vi "UHR-Fleezers Control (host) - 10.8MV_trial2.vi"() -> ()   [LabVIEW 2010] (continued)
          tunnel: [w5180] -> w5154
          tunnel: w5153 -> [w5180]
          tunnel: [w5179] -> w5147
          tunnel: w5146 -> [w5179]
          tunnel: [w5178] -> w5139
          tunnel: w5138 -> [w5178]
          tunnel: [w5184] -> w5155
          tunnel: w5154 -> [w5184]
          tunnel: [w5183] -> w5148
          tunnel: w5147 -> [w5183]
          tunnel: [w5182] -> w5140
          tunnel: w5139 -> [w5182]
          tunnel: w5155 -> [w5190]
          tunnel: w5148 -> [w5189]
          tunnel: [w5187] -> w5141
          tunnel: w5140 -> [w5187]
          tunnel: w5141 -> [w5191]
          frame #0 {
            n1099 = local read "Green Laser ON/Interlacing"() -> (w5159:bool)
            n1100 = local read "Green laser mode"() -> (w5158:enum32{"Laser ON", "Laser OFF", "Interlace"})
            n1101 = local read "Green FB On/Off"() -> (w5157:bool)
          }
          frame #1 {
            n1102 = property on="Green FB On/Off" class="Bool (strict)"("Val(Sgnl)"=FALSE ("Value (Signaling)")) -> ()  [unwired: 2 in, 2 out]
          }
          frame #2 {
            n1103 = property on="Green Laser ON/Interlacing" class="Bool (strict)"("Val(Sgnl)"=TRUE ("Value (Signaling)")) -> ()  [unwired: 2 in, 2 out]
            n1104 = property on="Flip Green Filter" class="Bool (strict)"("Val(Sgnl)"=TRUE ("Value (Signaling)")) -> ()  [unwired: 2 in, 2 out]
            n1105 = property on="Green laser mode" class="RadioBtnsControl (strict)"("Val(Sgnl)"=enum32{"Laser ON", "Laser OFF", "Interlace"}."Laser ON" ("Value (Signaling)")) -> ()  [unwired: 2 in, 2 out]
          }
          frame #3 {
            n1106 = Wait (ms)(milliseconds to wait=u32 500) -> ()  [unwired: 1 out]
          }
          frame #4 {
            n1107 = property on="Confocal Image" class="Bool (strict)"("Val(Sgnl)"=TRUE ("Value (Signaling)")) -> ()  [unwired: 2 in, 2 out]
          }
          frame #5 {
            n1108 = Wait (ms)(milliseconds to wait=u32 2000) -> ()  [unwired: 1 out]
          }
          frame #6 {
            n1109 = while {
              stop <- w5185 stop-if-true
              n1110 = local read "Saving..."() -> (w5186:bool)
              n1111 = Not(x=w5186) -> (.not. x?=w5185:bool)
            }
          }
          frame #7 {
            n1112 = property on="Flip Green Filter" class="Bool (strict)"("Val(Sgnl)"=TRUE ("Value (Signaling)")) -> ()  [unwired: 2 in, 2 out]
            n1113 = property on="Green Laser ON/Interlacing" class="Bool (strict)"("Val(Sgnl)"=w5190) -> ()  [unwired: 2 in, 2 out]
            n1114 = property on="Green laser mode" class="RadioBtnsControl (strict)"("Val(Sgnl)"=w5189) -> ()  [unwired: 2 in, 2 out]
          }
          frame #8 {
            n1115 = property on="Green FB On/Off" class="Bool (strict)"("Val(Sgnl)"=w5191) -> ()  [unwired: 2 in, 2 out]
          }
        }
      }
      event "Stop All": Value Change {
        n1116 = event-data() -> ()  [unwired: 1 in, 5 out]
        n1117 = local read "Stop All"() -> (w5192:bool)
      }
    }
    n1118 = node-c288() -> ()  [unwired: 1 in, 1 out]
  }
  n1119 = node-c288() -> (w76:T26)  [unwired: 4 out]
  n1120 = timed-loop "Mouse control: trap position (AOM deflection), set confocal spot from image" {
    tunnel: [w5194] -> w34
    tunnel: w24 -> [w5193]
    timing: w76 -> [_]
    timing-out: [_] -> w75
    stop <- w5194 stop-if-true
    n1121 = node-c288() -> ()  [unwired: 2 out]
    n1122 = event shown="[0] \"Pane\": Mouse Down" {
      selector: _ -> [_ _]
      dyn-events: _ -> [_ _]
      timeout: _ -> [_ _]
      tunnel: w5193 -> [w5197 _]
      event Mouse Down {
        n1123 = event-data() -> ("Time"=w5199:u32, "Coords"=w5198:T7, "Button"=w5200:u16)  [unwired: 6 out]
        n1124 = case shown="1" w5200 {
          tunnel: w5199 -> [_ _ w5303]
          tunnel: w5198 -> [_ w5237 w5301]
          tunnel: w5197 -> [_ _ w5299]
          frame 0, Default {
          }
          frame 1 {
            n1125 = property on="APD 2" class="ImageControl"() -> ("Displayed Image Position"=w5207:cluster{"Left":i32, "Top":i32})  [unwired: 2 in, 2 out]
            n1126 = property on="APD 1" class="ImageControl"() -> ("Displayed Image Position"=w5236:cluster{"Left":i32, "Top":i32})  [unwired: 2 in, 2 out]
            n1127 = property on="Detection Laser X" class="ImageControl"() -> ("Displayed Image Position"=w5233:cluster{"Left":i32, "Top":i32})  [unwired: 2 in, 2 out]
            n1128 = property on="Detection Laser Y" class="ImageControl"() -> ("Displayed Image Position"=w5232:cluster{"Left":i32, "Top":i32})  [unwired: 2 in, 2 out]
            n1129 = property on="APD 2" class="ImageControl"() -> ("Displayed Image Size"=w5206:cluster{"Width":u32, "Height":u32})  [unwired: 2 in, 2 out]
            n1130 = property on="APD 1" class="ImageControl"() -> ("Displayed Image Size"=w5234:cluster{"Width":u32, "Height":u32})  [unwired: 2 in, 2 out]
            n1131 = property on="Detection Laser X" class="ImageControl"() -> ("Displayed Image Size"=w5235:cluster{"Width":u32, "Height":u32})  [unwired: 2 in, 2 out]
            n1132 = property on="Detection Laser Y" class="ImageControl"() -> ("Displayed Image Size"=w5231:cluster{"Width":u32, "Height":u32})  [unwired: 2 in, 2 out]
            n1133 = Unbundle By Name(w5206) -> ("Width"=w5203:u32, "Height"=w5202:u32)
            n1134 = Unbundle By Name(w5207) -> ("Left"=w5205:i32, "Top"=w5204:i32)
            n1135 = Unbundle By Name(w5234) -> ("Width"=w5228:u32, "Height"=w5227:u32)
            n1136 = Unbundle By Name(w5235) -> ("Width"=w5224:u32, "Height"=w5223:u32)
            n1137 = Unbundle By Name(w5231) -> ("Width"=w5220:u32, "Height"=w5219:u32)
            n1138 = Unbundle By Name(w5236) -> ("Left"=w5230:i32, "Top"=w5229:i32)
            n1139 = Unbundle By Name(w5233) -> ("Left"=w5226:i32, "Top"=w5225:i32)
            n1140 = Unbundle By Name(w5232) -> ("Left"=w5222:i32, "Top"=w5221:i32)
            n1141 = Bundle("Left"=w5205, "Top"=w5204, "Width"=w5203, "Height"=w5202) -> (w5201:T35)  [unwired: 1 in]
            n1142 = Bundle("Left"=w5230, "Top"=w5229, "Width"=w5228, "Height"=w5227) -> (w5218:T35)  [unwired: 1 in]
            n1143 = Bundle("Left"=w5226, "Top"=w5225, "Width"=w5224, "Height"=w5223) -> (w5217:T35)  [unwired: 1 in]
            n1144 = Bundle("Left"=w5222, "Top"=w5221, "Width"=w5220, "Height"=w5219) -> (w5216:T35)  [unwired: 1 in]
            n1145 = Build Cluster Array(w5201, w5218, w5217, w5216) -> (w5215:T36)
            n1146 = for {
              tunnel: w5237 -> [w5248]
              tunnel: w5215 -> [w5249] mode=indexing
              shift-right: [w5246] -> w5213
              shift-left: TRUE -> [w5247]
              shift-right: [w5245] -> w5211
              shift-left: _ -> [w5241]
              shift-right: [w5244] -> w5210
              shift-left: _ -> [w5240]
              shift-right: [w5243] -> w5209
              shift-left: _ -> [w5239]
              shift-right: [w5242] -> w5208
              shift-left: _ -> [w5238]
              n1147 = case shown="True" w5247 {
                selector: w5247 -> [w5254 _]
                tunnel: w5249 -> [_ w5263]
                tunnel: w5248 -> [_ w5261]
                tunnel: [w5254 w5259] -> w5246
                tunnel: [w5253 w5258] -> w5245
                tunnel: [w5252 w5257] -> w5244
                tunnel: [w5251 w5256] -> w5243
                tunnel: [w5250 w5255] -> w5242
                tunnel: w5241 -> [w5253 _]
                tunnel: w5240 -> [w5252 _]
                tunnel: w5239 -> [w5251 _]
                tunnel: w5238 -> [w5250 _]
                frame False {
                }
                frame True {
                  n1148 = Unbundle(w5263) -> (w5262:T35)
                  n1149 = call "isclickinwindow.vi"("Image Param"=w5262, "Point32"=w5261) -> ("4 Y"=w5255:i32, "3 Height"=w5256:i32, "2 X"=w5257:i32, "1 Width"=w5258:i32, "In image?"=w5260:bool)  [unwired: 1 in]
                  n1150 = Not(x=w5260) -> (.not. x?=w5259:bool)
                }
              }
            }
            n1151 = Not(x=w5213) -> (.not. x?=w5212:bool)
            n1152 = case shown="True" w5212 {
              tunnel: w5210 -> [_ w5276]
              tunnel: w5208 -> [_ w5275]
              tunnel: w5211 -> [_ w5274]
              tunnel: w5209 -> [_ w5273]
              frame False {
              }
              frame True {
                w5269 = FALSE ("Get Point")
                n1153 = local read "Scan lines (y)"() -> (w5278:u64)
                n1154 = local read "Actual MCL Inc (V)"() -> (w5270:dbl)
                n1155 = local read "Scan steps (MCL)"() -> (w5277:u64)
                n1156 = Divide "Y Pix/step"(x=w5273, y=w5278) -> (x/y=w5285:dbl)
                n1157 = Divide "Y V/pix"(x=w5270, y=w5285) -> (x/y=w5284:dbl)
                n1158 = Divide "Y half step offset"(x=w5270, y=2.0) -> (x/y=w5286:dbl)
                n1159 = Divide "X pix/step"(x=w5274, y=w5277) -> (x/y=w5283:dbl)
                n1160 = Negate(x=w5286) -> (-x=w5287:dbl)
                n1161 = local read "Initial Y"() -> (w5293:dbl)
                n1162 = Multiply(x=w5275, y=w5284) -> (x*y=w5294:dbl)
                n1163 = Divide "X half step offset"(x=w5270, y=2.0) -> (x/y=w5280:dbl)
                n1164 = Divide "X V/pix"(x=w5270, y=w5283) -> (x/y=w5282:dbl)
                n1165 = Multiply(x=w5270, y=w5277) -> (x*y=w5289:dbl)
                n1166 = Compound Arithmetic op=ADD(w5287, w5294, w5293) -> (w5271:dbl)
                "Pointer Y (V)" <- w5271
                n1167 = Multiply(x=w5282, y=w5276) -> (x*y=w5291:dbl)
                n1168 = Negate(x=w5280) -> (-x=w5279:dbl)
                n1169 = local read "Initial X"() -> (w5292:dbl)
                n1170 = Negate(x=w5291) -> (-x=w5290:dbl)
                n1171 = Compound Arithmetic op=ADD(w5279, w5289, w5292, w5290) -> (w5272:dbl)
                "Pointer X (V)" <- w5272
                n1172 = Or(x="Set X Only", y="Set Confocal Spot (X-Y)") -> (x .or. y?=w5265:bool)
                n1173 = Or(x="Set Confocal Spot (X-Y)", y="Set Y Only") -> (x .or. y?=w5264:bool)
                n1174 = case shown="True" w5265 {
                  tunnel: w5272 -> [_ w5295]
                  frame False {
                  }
                  frame True {
                    n1175 = property on="AO2" class="Slide (strict)"("Val(Sgnl)"=w5295) -> ()  [unwired: 2 in, 2 out]
                  }
                }
                n1176 = case shown="True" w5264 {
                  tunnel: w5271 -> [_ w5296]
                  frame False {
                  }
                  frame True {
                    n1177 = property on="AO1" class="Slide (strict)"("Val(Sgnl)"=w5296) -> ()  [unwired: 2 in, 2 out]
                  }
                }
                n1178 = local write "Set Confocal Spot (X-Y)"(w5269) -> ()
                n1179 = local write "Set X Only"(w5269) -> ()
                n1180 = local write "Set Y Only"(w5269) -> ()
              }
            }
          }
          frame 3 {
            n1181 = local read "BD 2 Frequency 1 (MHz)"() -> (w5297:dbl)
            n1182 = local read "BD 1 Frequency 1 (MHz)"() -> (w5298:dbl)
            n1183 = local write "Manipulating Trap"(TRUE ("Manipulating Trap")) -> ()
            n1184 = local write "Coords"(T7 {"Horizontal"=0, "Vertical"=0} ("Coords")) -> ()
            n1185 = while {
              tunnel: w5303 -> [w5308]
              tunnel: w5301 -> [w5307]
              tunnel: w5299 -> [w5306]
              tunnel: w5298 -> [w5305]
              tunnel: w5297 -> [w5304]
              stop <- w5309 stop-if-true
              n1186 = event shown="[0] \"Pane\": Mouse Move" {
                selector: _ -> [_ _]
                dyn-events: _ -> [_ _]
                timeout: _ -> [_ _]
                tunnel: ["Force Manip Abort" w5373] -> w5309
                tunnel: w5308 -> [w5316 _]
                tunnel: w5307 -> [w5314 _]
                tunnel: w5306 -> [w5313 _]
                tunnel: w5305 -> [w5312 _]
                tunnel: w5304 -> [w5311 _]
                event Mouse Move {
                  n1187 = event-data() -> ("Time"=w5317:u32, "Coords"=w5318:T7)  [unwired: 3 out]
                  n1188 = Less?(x=w5317, y=w5316) -> (x < y?=w5315:bool)
                  n1189 = case "Makes sure old motion events prior to mouse click aren't used" shown="False" w5315 {
                    tunnel: w5318 -> [w5360 _]
                    tunnel: w5314 -> [w5361 _]
                    tunnel: w5313 -> [w5338 _]
                    tunnel: w5312 -> [w5334 _]
                    tunnel: w5311 -> [w5333 _]
                    frame False {
                      n1190 = Subtract(x=w5360, y=w5361) -> (x-y=w5359:T7)
                      "Coords" <- w5359
                      n1191 = local read "Y RF Frequency Limits (MHz)"() -> (w5319:T16)
                      n1192 = To Double Precision Float(number=w5359) -> (double precision float=w5358:cluster{"Horizontal":dbl, "Vertical":dbl})
                      n1193 = Multiply(x=cluster{"Horizontal":dbl, "Vertical":dbl} {"Horizontal"=-1.0, "Vertical"=1.0}, y="Manipulation Scaling") -> (x*y=w5354:cluster{"Horizontal":dbl, "Vertical":dbl})
                      n1194 = local read "X RF Frequency Limits (MHz)"() -> (w5320:T16)
                      n1195 = Multiply(x=w5358, y=w5354) -> (x*y=w5356:cluster{"Horizontal":dbl, "Vertical":dbl})
                      n1196 = Unbundle By Name(w5356) -> ("Horizontal"=w5351:dbl, "Vertical"=w5355:dbl)
                      n1197 = Unbundle By Name(w5319) -> ("Maximum"=w5322:dbl, "Minimum"=w5321:dbl)
                      n1198 = Boolean To (0,1)(Boolean="Manip. X?") -> (0, 1=w5349:i16)
                      n1199 = Boolean To (0,1)(Boolean="Manip. Y?") -> (0, 1=w5346:i16)
                      n1200 = local read "BD 1 Frequency 2 (MHz)"() -> (w5336:dbl)
                      n1201 = Multiply(x=w5355, y=w5346) -> (x*y=w5348:dbl)
                      n1202 = Multiply(x=w5349, y=w5351) -> (x*y=w5352:dbl)
                      n1203 = local read "BD 2 Frequency 2 (MHz)"() -> (w5335:dbl)
                      n1204 = Unbundle By Name(w5320) -> ("Maximum"=w5324:dbl, "Minimum"=w5323:dbl)
                      n1205 = Add(x=w5333, y=w5348) -> (x+y=w5326:dbl)
                      n1206 = Add(x=w5334, y=w5352) -> (x+y=w5328:dbl)
                      n1207 = In Range and Coerce(upper limit=w5324, x=w5328, lower limit=w5323) -> (coerced(x)=w5327:dbl)  [unwired: 1 out]
                      n1208 = In Range and Coerce(upper limit=w5322, x=w5326, lower limit=w5321) -> (coerced(x)=w5325:dbl)  [unwired: 1 out]
                      n1209 = Subtract(x=w5327, y=w5336) -> (x-y=w5345:dbl)
                      n1210 = Subtract(x=w5325, y=w5335) -> (x-y=w5344:dbl)
                      n1211 = Square(x=w5345) -> (x^2=w5343:dbl)
                      n1212 = Square(x=w5344) -> (x^2=w5342:dbl)
                      n1213 = Add(x=w5343, y=w5342) -> (x+y=w5341:dbl)
                      n1214 = Square Root(x=w5341) -> (sqrt(x)=w5337:dbl)
                      n1215 = In Range and Coerce(upper limit="Limit Max (MHz)", x=w5337, lower limit="Limit Min (MHz)") -> (In Range?=w5330:bool)  [unwired: 1 out]
                      n1216 = Not(x="Limits Enable") -> (.not. x?=w5329:bool)
                      n1217 = Or(x=w5330, y=w5329) -> (x .or. y?=w5331:bool)
                      n1218 = case shown="True" w5331 {
                        tunnel: w5338 -> [_ w5371]
                        tunnel: w5337 -> [_ w5362]
                        tunnel: w5327 -> [_ w5369]
                        tunnel: w5336 -> [_ w5368]
                        tunnel: w5325 -> [_ w5367]
                        tunnel: w5335 -> [_ w5366]
                        tunnel: w5320 -> [_ w5364]
                        tunnel: w5319 -> [_ w5363]
                        frame False {
                        }
                        frame True {
                          n1219 = local read "BD 1 Frequency 3 (MHz)"() -> (w5370:dbl)
                          n1220 = local read "BD 2 Frequency 3 (MHz)"() -> (w5365:dbl)
                          n1221 = local write "Trap Delta (MHz)"(w5362) -> ()
                          n1222 = property on="Initial delta (MHz)" class="DigNum (strict)"("Val(Sgnl)"=w5362) -> ()  [unwired: 2 in, 2 out]
                          n1223 = call "set RF board frequency - interlace.vi"("Board 2 Frequency Limits"=w5363, "Board 1 Frequency Limits"=w5364, "FPGA VI Reference In"=w5371, "Board 2 Frequency 3 (MHz)"=w5365, "Board 1 Frequency 3 (MHz)"=w5370, "Board 2 Frequency 2 (MHz)"=w5366, "Board 2 Frequency 1 (MHz)"=w5367, "Board 1 Frequency 2 (MHz)"=w5368, "Board 1 Frequency 1  (MHz)"=w5369) -> ()  [unwired: 1 in, 2 out]
                          n1224 = local write "BD 2 Frequency 1 (MHz)"(w5367) -> ()
                          n1225 = local write "BD 1 Frequency 1 (MHz)"(w5369) -> ()
                        }
                      }
                    }
                    frame True {
                    }
                  }
                }
                event Mouse Up {
                  n1226 = event-data() -> ("Button"=w5372:u16)  [unwired: 8 out]
                  n1227 = case shown="3" w5372 {
                    tunnel: [FALSE TRUE] -> w5373
                    frame 0, Default {
                    }
                    frame 3 {
                      n1228 = local write "Manipulating Trap"(FALSE ("Manipulating Trap")) -> ()
                    }
                  }
                }
              }
            }
          }
        }
      }
      event Mouse Move {
        n1229 = event-data() -> ()  [unwired: 6 out]
      }
    }
    n1230 = local read "Stop All"() -> (w5194:bool)
    n1231 = node-c288() -> ()  [unwired: 2 out]
  }
  n1232 = node-c288(i64 1 ("Period"), 1 ("Processor")) -> (w164:T26)  [unwired: 2 out]
  n1233 = timed-loop "Acquire Data" {
    tunnel: w24 -> [w5631]
    tunnel: w40 -> [w5630]
    tunnel: [w5661] -> w33
    tunnel: [w5655] -> w32
    timing: w164 -> [_]
    timing-out: [_] -> w163
    tunnel: w59 -> [w5459]
    stop <- "Stop All" stop-if-true
    (unwired) u32 0 ("Number of Elements")
    w5446 = "NI_ChannelName" ("name")
    n1234 = node-c288() -> ()  [unwired: 2 out]
    n1235 = First Call?() -> (First Call?: T/F=w5412:bool)
    n1236 = Or(x="Reset", y=w5412) -> (x .or. y?=w5413:bool)
    n1237 = case "Reset data stream" shown="True" w5413 {
      tunnel: w5631 -> [w5749 w5757]
      tunnel: w5630 -> [w5748 w5756]
      tunnel: [w5749 w5751] -> w5626
      tunnel: [w5748 w5750] -> w5625
      frame False {
      }
      frame True {
        w5754 = TRUE ("AI to FIFO")
        n1238 = local write "Overflow (data lost)"(FALSE ("Overflow (data lost)")) -> ()
        n1239 = call "reset FPGA DMA.vi"("error in"=w5756, "FPGA VI Reference In"=w5757) -> ("error out"=w5752:errorcluster, "FPGA VI Reference Out"=w5753:T19)
        n1240 = xnode "Read/Write Control"("FPGA VI Reference In"=w5753, "error in"=w5752, "AI to FIFO"=w5754, "APD to FIFO"=w5754) -> ("FPGA VI Reference Out"=w5751:T19, "error out"=w5750:errorcluster)
      }
    }
    n1241 = Or(x="Start AOD Scan", y="Trap Raster Scan") -> (x .or. y?=w5576:bool)
    n1242 = case "Start AOM raster scan" shown="True" w5576 {
      tunnel: w5626 -> [w7357 w7367]
      tunnel: w5625 -> [w7356 w7366]
      tunnel: [w7357 w7360] -> w5624
      tunnel: [w7356 w7359] -> w5623
      frame False {
      }
      frame True {
        n1243 = case shown="True" "Restart DMA? (AOD)" {
          tunnel: [w7778 w7780] -> w7361
          tunnel: [w7777 w7779] -> w7362
          tunnel: w7367 -> [w7778 w7782]
          tunnel: w7366 -> [w7777 w7781]
          frame False {
          }
          frame True {
            n1244 = local write "Overflow (data lost)"(FALSE ("Overflow (data lost)")) -> ()
            n1245 = call "reset FPGA DMA.vi"("error in"=w7781, "FPGA VI Reference In"=w7782) -> ("error out"=w7779:errorcluster, "FPGA VI Reference Out"=w7780:T19)
          }
        }
        n1246 = local write "Trap Raster Scan"(FALSE ("Trap Raster Scan")) -> ()
        n1247 = case shown="False" "Move MCL Also?" {
          tunnel: w7362 -> [w7370 w7479]
          tunnel: w7361 -> [w7371 w7480]
          tunnel: [w7369 w7483] -> w7360
          tunnel: [w7368 w7482] -> w7359
          frame False {
            w7372 = TRUE ("AI to FIFO")
            n1248 = xnode "Read/Write Control"("FPGA VI Reference In"=w7371, "error in"=w7370, "AI to FIFO"=w7372, "APD to FIFO"=w7372, "Start scan"=w7372) -> ("FPGA VI Reference Out"=w7369:T19, "error out"=w7368:errorcluster)
          }
          frame True {
            w7476 = FALSE ("1D or 2D Scan?")
            w7481 = TRUE ("AI to FIFO")
            # "Count for MCL loop"
            # "N total cycles"
            # "N steps"
            # "V_int"
            n1249 = local read "Scan Range (nm)"() -> (w7458:dbl)
            n1250 = local read "Number of F/B Scans (AOD)"() -> (w7475:u16)
            n1251 = Sign(1:w7458) -> (0:w7457:dbl)
            n1252 = Compound Arithmetic op=MULTIPLY(w7458, "MCL Step Position Ratio", "MCL/AOM Scale Tweak") -> (w7462:dbl)
            n1253 = Negate(x=w7457) -> (-x=w7454:dbl)
            n1254 = Multiply(x=w7454, y="MCL Step Increment (V_int)") -> (x*y=w7456:dbl)
            n1255 = Divide(x=w7462, y="MCL X Cal (nm/V)") -> (x/y=w7468:dbl)
            n1256 = Multiply(x=32767.0 ("y"), y=w7468) -> (x*y=w7474:dbl)
            n1257 = local read "Total Counts (ticks)"() -> (w7459:u32)
            n1258 = local read "Cycles/step (AOD)"() -> (w7470:u64)
            n1259 = local read "Scan steps (AOD)"() -> (w7471:u64)
            n1260 = Divide(x=w7474, y=10.0) -> (x/y=w7467:dbl)
            n1261 = Divide(x=w7467, y="MCL Step Increment (V_int)") -> (x/y=w7465:dbl)
            n1262 = Absolute Value(x=w7465) -> (abs(x)=w7453:dbl)
            n1263 = Compound Arithmetic op=MULTIPLY(w7471, w7470, w7459) -> (w7466:u64)
            n1264 = local write "wait to reset values"(w7481) -> ()
            n1265 = local write "MCL Scanning"(w7481) -> ()
            n1266 = Divide(x=w7466, y=w7453) -> (x/y=w7463:dbl)
            "MCL Count" <- w7463
            n1267 = xnode "Read/Write Control"("FPGA VI Reference In"=w7480, "error in"=w7479, "Scan steps (MCL)"=w7453, "Number of scans (MCL)"=w7475, "Cycles per step (MCL)"=u64 1, "Scan freq.  increment (MCL)"=w7456, "1D or 2D Scan?"=w7476, "MCL Scan Axis"=w7476, "Cont. Scan (MCL)"=w7476, "MCL count"=w7463) -> ("FPGA VI Reference Out"=w7478:T19, "error out"=w7477:errorcluster)
            n1268 = xnode "Read/Write Control"("FPGA VI Reference In"=w7478, "error in"=w7477, "AI to FIFO"=w7481, "APD to FIFO"=w7481, "Start scan"=w7481, "Start scan (MCL)"=w7481) -> ("FPGA VI Reference Out"=w7483:T19, "error out"=w7482:errorcluster)
          }
        }
        "Raster Scanning..." <- TRUE ("Scanning...")
      }
    }
    n1269 = And(x="Save scans", y=w5576) -> (x .and. y?=w5622:bool)
    n1270 = Compound Arithmetic op=OR("Start MCL Scan", "Confocal Image", "Confocal Linescan") -> (w5574:bool)
    n1271 = And(x="Save Data (MCL)", y=w5574) -> (x .and. y?=w5621:bool)
    n1272 = case "Start MCL raster scan" shown="True" w5574 {
      tunnel: w5624 -> [w6634 w6649]
      tunnel: w5623 -> [w6633 w6648]
      tunnel: [w6634 w6644] -> w5381
      tunnel: [w6633 w6643] -> w5380
      tunnel: [FALSE w6642] -> w5607
      tunnel: "Start MCL Scan" -> [_ w6637]
      tunnel: "Confocal Image" -> [_ w6636]
      tunnel: "Confocal Linescan" -> [_ _]
      frame False {
      }
      frame True {
        w6642 = TRUE
        n1273 = case shown="True" "Restart DMA? (MCL)" {
          tunnel: [w6894 w6896] -> w6647
          tunnel: [w6893 w6895] -> w6646
          tunnel: w6649 -> [w6894 w6899]
          tunnel: w6648 -> [w6893 w6898]
          frame False {
          }
          frame True {
            n1274 = call "reset FPGA DMA.vi"("error in"=w6898, "FPGA VI Reference In"=w6899) -> ("error out"=w6895:errorcluster, "FPGA VI Reference Out"=w6896:T19)
            n1275 = local write "Overflow (data lost)"(FALSE ("Overflow (data lost)")) -> ()
          }
        }
        n1276 = case shown="False" w6637 {
          selector: w6637 -> [_ w6653]
          tunnel: w6636 -> [w6652 _]
          tunnel: [w6652 w6653] -> w6635
          frame False {
            n1277 = property on="2D or 1D Scan" class="Bool (strict)"("Val(Sgnl)"=w6652) -> ()  [unwired: 2 in, 2 out]
            n1278 = property on="Confocal Image" class="Bool (strict)"("Value"=FALSE ("Start Confocal Map")) -> ()  [unwired: 2 in, 2 out]
          }
          frame True {
          }
        }
        n1279 = local write "MCL Scanning"(w6642) -> ()
        n1280 = local read "AO1"() -> (w6639:dbl)
        n1281 = local read "AO2"() -> (w6638:dbl)
        n1282 = case shown="True" "Center Scan" {
          tunnel: w6647 -> [w6660 w6772]
          tunnel: w6646 -> [w6659 w6771]
          tunnel: [w6658 w6770] -> w6644
          tunnel: [w6657 w6769] -> w6643
          tunnel: [w6655 w6756] -> w6641
          tunnel: [w6654 w6755] -> w6640
          tunnel: w6639 -> [w6655 w6761]
          tunnel: w6638 -> [w6654 w6764]
          tunnel: w6635 -> [_ _]
          frame False {
            w6656 = TRUE ("AI to FIFO")
            n1283 = xnode "Read/Write Control"("FPGA VI Reference In"=w6660, "error in"=w6659, "AI to FIFO"=w6656, "APD to FIFO"=w6656, "Start scan (MCL)"=w6656) -> ("FPGA VI Reference Out"=w6658:T19, "error out"=w6657:errorcluster)
          }
          frame True {
            w6768 = TRUE ("AI to FIFO")
            n1284 = local read "Scan steps (MCL)"() -> (w6747:u64)
            n1285 = local read "Scan lines (y)"() -> (w6743:u64)
            n1286 = local read "Fast Scan Dir"() -> (w6754:bool)
            n1287 = local read "Actual MCL Inc (V)"() -> (w6744:dbl)
            n1288 = Decrement(x=w6743) -> (x-1=w6742:u64)
            n1289 = Decrement(x=w6747) -> (x-1=w6746:u64)
            n1290 = Multiply(x=w6744, y=w6742) -> (x*y=w6741:dbl)
            n1291 = Divide(x=w6741, y=2.0) -> (x/y=w6751:dbl)
            n1292 = Multiply(x=w6744, y=w6746) -> (x*y=w6745:dbl)
            n1293 = Divide(x=w6745, y=2.0) -> (x/y=w6750:dbl)
            n1294 = Select(t=w6750, s=w6754, f=w6751) -> (s? t:f=w6749:dbl)
            n1295 = Select(t=w6751, s=w6754, f=w6750) -> (s? t:f=w6753:dbl)
            n1296 = Subtract(x=w6761, y=w6753) -> (x-y=w6752:dbl)
            n1297 = Subtract(x=w6764, y=w6749) -> (x-y=w6748:dbl)
            n1298 = local read "2D or 1D Scan"() -> (w6766:bool)
            n1299 = Not(x=w6754) -> (.not. x?=w6760:bool)
            n1300 = Not(x=w6766) -> (.not. x?=w6762:bool)
            n1301 = And(x=w6754, y=w6762) -> (x .and. y?=w6763:bool)
            n1302 = And(x=w6762, y=w6760) -> (x .and. y?=w6765:bool)
            n1303 = Select(t=w6764, s=w6765, f=w6748) -> (s? t:f=w6755:dbl)
            n1304 = Select(t=w6761, s=w6763, f=w6752) -> (s? t:f=w6756:dbl)
            n1305 = call "Volt to I16.vi"("Voltage In"=w6756) -> ("I16 Voltage Out"=w6759:i16)
            n1306 = call "Volt to I16.vi"("Voltage In"=w6755) -> ("I16 Voltage Out"=w6758:i16)
            n1307 = xnode "Read/Write Control"("FPGA VI Reference In"=w6772, "error in"=w6771, "AI to FIFO"=w6768, "APD to FIFO"=w6768, "Start scan (MCL)"=w6768, "AO1"=w6759, "AO2"=w6758) -> ("FPGA VI Reference Out"=w6770:T19, "error out"=w6769:errorcluster)
          }
        }
        "Initial Y" <- w6641
        "Initial X" <- w6640
        "wait to reset values" <- w6642
      }
    }
    n1308 = local read "Trap Pos Elements/DMA read"() -> (w5455:u32)
    n1309 = local read "Trap AI Elements/DMA read"() -> (w5379:u32)
    n1310 = local read "APD Elements/DMA read"() -> (w5498:u32)
    n1311 = local read "Trap AI FIFO Depth"() -> (w5671:u32)
    n1312 = xnode "Invoke Method"("FPGA VI Reference In"=w5381, "error in"=w5380, "Number of Elements"=w5455, "Timeout (ms)"=-1) -> ("Data"=w5419:u16[], "Elements Remaining"=→"Trap Pos FIFO El Remaining":u32)  [unwired: 2 out]
    n1313 = xnode "Invoke Method"("FPGA VI Reference In"=w5381, "error in"=w5380, "Number of Elements"=w5379, "Timeout (ms)"=-1 ("Timeout")) -> ("FPGA VI Reference Out"=w5383:T19, "error out"=w5382:errorcluster, "Data"=w5378:i16[], "Elements Remaining"=w5384:u32)
    "Trap AI FIFO El. Rem." <- w5384
    n1314 = xnode "Get APD Data"("FPGA VI Reference In"=w5381, "error in"=w5380, "Number of Elements"=w5498, "Timeout (ms)"=-1) -> ("Data"=w5497:u32[], "Elements Remaining"=→"APD FIFO Elements Remaining":u32)  [unwired: 2 out]
    n1315 = Subtract(x=w5671, y=w5379) -> (x-y=w5670:u32)
    n1316 = Decimate 1D Array(w5419) -> (w5416:u16[], w5418:u16[], w5417:u16[])
    n1317 = Divide(x=w5384, y=w5670) -> (x/y=w5669:dbl)
    "Buffer Status" <- w5669
    n1318 = To Unsigned Long Integer(number=w5416) -> (unsigned 32bit integer=w5415:u32[])
    n1319 = Join Numbers(hi=w5418, lo=w5417) -> ((hi.lo)=w5414:u32[])
    n1320 = Equal?(x=w5669, y=1.0) -> (x = y?=w5667:bool)
    n1321 = Join Numbers(hi=w5415, lo=w5414) -> ((hi.lo)=w5408:u64[])
    n1322 = call "IR AOM word to freq - vec.vi"("Frequency Word In (double vec)"=w5408) -> ("Frequency Out"=w5454:dbl[])
    n1323 = case "Alert buffer overflow" shown="True" w5667 {
      frame False {
      }
      frame True {
        n1324 = call <vilib>:"Beep.vi"() -> ()  [unwired: 3 in, 9 out]
        "Overflow (data lost)" <- TRUE ("Overflow (data lost)")
      }
    }
    n1325 = Decimate 1D Array(w5454) -> (w5453:dbl[], w5452:dbl[])
    n1326 = Array Size(array=w5378) -> (size(s)=→"Waveform Chart":i32)
    n1327 = Build Array(w5453, w5452) -> (w5451:dbl[][])
    n1328 = local read "Trap Sets"() -> (w5535:u32)
    n1329 = case "Deinterlace trap data, average down PSD" shown="2" w5535 {
      tunnel: w5378 -> [w6929 w6994]
      tunnel: [w6926 w6991] -> w5528
      tunnel: [w6929 w6993] -> w5411
      tunnel: "Detector Type" -> [w6928 w6989]
      tunnel: [w6927 w6992] -> w5527
      tunnel: [w6925 w6990] -> w5642
      frame 1, Default {
        n1330 = Divide(x=w6929, y=3276.7) -> (x/y=w6930:dbl[])
        n1331 = Decimate 1D Array(w6930) -> (w6939:dbl[], w6938:dbl[], w6937:dbl[], w6936:dbl[], w6935:dbl[], w6934:dbl[], w6933:dbl[], w6932:dbl[])
        n1332 = case shown="\"IR-QPD + PSD + FB-QPD position\"" w6928 {
          tunnel: w6939 -> [w6963 w6988]
          tunnel: w6938 -> [w6962 w6987]
          tunnel: w6937 -> [w6947 w6965]
          tunnel: w6936 -> [w6948 w6975]
          tunnel: w6935 -> [w6961 w6986]
          tunnel: w6934 -> [w6960 w6985]
          tunnel: w6933 -> [w6944 w6966]
          tunnel: w6932 -> [w6943 w6964]
          tunnel: [w6942 w6972] -> w6927
          tunnel: [w6941 w6971] -> w6926
          tunnel: [w6940 w6970] -> w6925
          frame "IR-QPD + PSD + FB-QPD", Default {
            w6940 = 0  # Channel pattern
            n1333 = Divide(x=w6963, y=w6948) -> (x/y=w6950:dbl[])
            n1334 = Divide(x=w6962, y=w6948) -> (x/y=w6949:dbl[])
            n1335 = Divide(x=w6961, y=w6944) -> (x/y=w6946:dbl[])
            n1336 = Divide(x=w6960, y=w6943) -> (x/y=w6945:dbl[])
            n1337 = Build Array(w6950, w6949, w6948, w6947, w6946, w6945, w6944, w6943) -> (w6941:dbl[][])
            n1338 = Bundle("T1 Y", "T1 X", "T1 Sum", "FB Sum", "PSD Y", "PSD X", "PSD Y Sum", "PSD X Sum") -> (w6959:T44)  [unwired: 1 out]
            n1339 = Cluster To Array(cluster=w6959) -> (array=w6942:string[])
          }
          frame "IR-QPD + PSD + FB-QPD position" {
            w6970 = 3  # Channel pattern
            n1340 = Negate(x=w6966) -> (-x=w6967:dbl[])
            n1341 = Divide(x=w6988, y=w6975) -> (x/y=w6977:dbl[])
            n1342 = Divide(x=w6987, y=w6975) -> (x/y=w6976:dbl[])
            n1343 = Divide(x=w6986, y=w6966) -> (x/y=w6974:dbl[])
            n1344 = Divide(x=w6985, y=w6967) -> (x/y=w6973:dbl[])
            n1345 = Build Array(w6977, w6976, w6975, w6964, w6965, w6974, w6973, w6966) -> (w6971:dbl[][])
            n1346 = Bundle("T1 Y", "T1 X", "T1 Sum", "FB X", "FB Sum", "PSD Y", "PSD X", "PSD Y Sum") -> (w6984:T44)  [unwired: 1 out]
            n1347 = Cluster To Array(cluster=w6984) -> (array=w6972:string[])
          }
        }
      }
      frame 2 {
        n1348 = case shown="\"UCB Fleezers 052511\"" w6989 {
          tunnel: w6994 -> [w7056 w7123 w7151 w7258]
          tunnel: [w6995 w7115 w7146 w7189] -> w6993
          tunnel: [w7022 w7106 w7148 w7236] -> w6992
          tunnel: [w7021 w7070 w7125 w7203] -> w6991
          tunnel: [w7015 w7105 w7188 w7234] -> w6990
          frame "IR-QPD + PSD + FB-QPD", Default {
            w7015 = 1  # Channel pattern
            # "time average x2 the 4th signal and the 4 psd signals (detection laser)"
            # "deinterlace 3 signals from qpd"
            n1349 = Decimate 1D Array(w7056) -> (w7055:i16[], w7054:i16[], w7020:i16[], w7053:i16[], w7043:i16[], w7041:i16[], w7040:i16[], w7038:i16[])
            n1350 = call "downsample 1D array - double.vi"("Ave N"=2.0, "Array In"=w7043) -> ("Array Out"=w7042:dbl[])  [unwired: 1 out]
            n1351 = call "downsample 1D array - double.vi"("Ave N"=2.0, "Array In"=w7038) -> ("Array Out"=w7037:dbl[])  [unwired: 1 out]
            n1352 = call "downsample 1D array - double.vi"("Ave N"=2.0, "Array In"=w7040) -> ("Array Out"=w7039:dbl[])  [unwired: 1 out]
            n1353 = call "downsample 1D array - double.vi"("Ave N"=2.0, "Array In"=w7041) -> ("Array Out"=w7023:dbl[])  [unwired: 1 out]
            n1354 = Decimate 1D Array(w7055) -> (w7052:i16[], w7024:i16[])
            n1355 = Decimate 1D Array(w7054) -> (w7051:i16[], w7049:i16[])
            n1356 = Decimate 1D Array(w7053) -> (w7050:i16[], w7048:i16[])
            n1357 = Decimate 1D Array(w7020) -> (w7019:i16[], w7018:i16[])
            n1358 = Interleave 1D Arrays(w7052, w7051, w7050, w7024, w7049, w7048, w7019, w7018, w7042, w7023, w7039, w7037) -> (w7036:dbl[])
            n1359 = To Word Integer(number=w7036) -> (16bit integer=w6995:i16[])
            n1360 = Divide(x=w7036, y=3276.7) -> (x/y=w7035:dbl[])
            n1361 = Decimate 1D Array(w7035) -> (w7034:dbl[], w7033:dbl[], w7032:dbl[], w7031:dbl[], w7030:dbl[], w7029:dbl[], w7017:dbl[], w7016:dbl[], w7028:dbl[], w7027:dbl[], w7026:dbl[], w7025:dbl[])
            n1362 = Divide(x=w7034, y=w7032) -> (x/y=w7002:dbl[])
            n1363 = Divide(x=w7033, y=w7032) -> (x/y=w7001:dbl[])
            n1364 = Divide(x=w7031, y=w7029) -> (x/y=w7000:dbl[])
            n1365 = Divide(x=w7030, y=w7029) -> (x/y=w6999:dbl[])
            n1366 = Divide(x=w7028, y=w7026) -> (x/y=w6998:dbl[])
            n1367 = Divide(x=w7027, y=w7025) -> (x/y=w6997:dbl[])
            n1368 = Bundle("T1 Y", "T1 X", "T1 Sum", "T2 Y", "T2 X", "T2 Sum", "T1 FB Sum", "T2 FB Sum", "PSD Y", "PSD X", "PSD Y Sum", "PSD X Sum") -> (w7003:T45)  [unwired: 1 out]
            n1369 = Build Array(w7002, w7001, w7032, w7000, w6999, w7029, w7017, w7016, w6998, w6997, w7026, w7025) -> (w7021:dbl[][])
            n1370 = Cluster To Array(cluster=w7003) -> (array=w7022:string[])
          }
          frame "IR-QPD + PSD + FB-QPD X position" {
            w7105 = 2  # Channel pattern
            # "convert\nADC numbers\nto volts"
            # "time average x2 the 3 psd signals (detection laser)"
            # "deinterlace 3 signals from qpds"
            n1371 = Decimate 1D Array(w7123) -> (w7122:i16[], w7121:i16[], w7058:i16[], w7059:i16[], w7068:i16[], w7065:i16[], w7062:i16[], w7093:i16[])
            n1372 = Decimate 1D Array(w7122) -> (w7120:i16[], w7107:i16[])
            n1373 = call "downsample 1D array - I16.vi"("Ave N"=2.0, "Array In"=w7068) -> ("Array Out"=w7066:i16[])  [unwired: 1 in]
            n1374 = call "downsample 1D array - I16.vi"("Ave N"=2.0, "Array In"=w7065) -> ("Array Out"=w7063:i16[])  [unwired: 1 in]
            n1375 = Decimate 1D Array(w7121) -> (w7119:i16[], w7117:i16[])
            n1376 = Decimate 1D Array(w7059) -> (w7118:i16[], w7116:i16[])
            n1377 = Decimate 1D Array(w7093) -> (w7092:i16[], w7090:i16[])
            n1378 = Decimate 1D Array(w7058) -> (w7091:i16[], w7089:i16[])
            n1379 = call "downsample 1D array - I16.vi"("Ave N"=2.0, "Array In"=w7062) -> ("Array Out"=w7060:i16[])  [unwired: 1 in]
            n1380 = Interleave 1D Arrays(w7120, w7119, w7118, w7107, w7117, w7116, w7092, w7091, w7090, w7089, w7066, w7063, w7060) -> (w7115:i16[])
            n1381 = Divide(x=w7115, y=3276.7) -> (x/y=w7114:dbl[])
            n1382 = Decimate 1D Array(w7114) -> (w7113:dbl[], w7112:dbl[], w7111:dbl[], w7110:dbl[], w7109:dbl[], w7108:dbl[], w7081:dbl[], w7079:dbl[], w7078:dbl[], w7076:dbl[], w7075:dbl[], w7074:dbl[], w7071:dbl[])
            n1383 = Divide(x=w7113, y=w7111) -> (x/y=w7097:dbl[])
            n1384 = Divide(x=w7112, y=w7111) -> (x/y=w7096:dbl[])
            n1385 = Divide(x=w7110, y=w7108) -> (x/y=w7095:dbl[])
            n1386 = Divide(x=w7109, y=w7108) -> (x/y=w7094:dbl[])
            n1387 = Divide(x=w7081, y=w7079) -> (x/y=w7080:dbl[])
            n1388 = Divide(x=w7078, y=w7076) -> (x/y=w7077:dbl[])
            n1389 = Divide(x=w7075, y=w7071) -> (x/y=w7073:dbl[])
            n1390 = Negate(x=w7071) -> (-x=w7069:dbl[])
            n1391 = Divide(x=w7074, y=w7069) -> (x/y=w7072:dbl[])
            n1392 = Bundle("T1 Y", "T1 X", "T1 Sum", "T2 Y", "T2 X", "T2 Sum", "T1 FB X", "T1 FB Sum", "T2 FB X", "T2 FB Sum", "PSD Y", "PSD X", "PSD Y Sum") -> (w7098:T46)  [unwired: 1 out]
            n1393 = Build Array(w7097, w7096, w7111, w7095, w7094, w7108, w7080, w7079, w7077, w7076, w7073, w7072, w7071) -> (w7070:dbl[][])
            n1394 = Cluster To Array(cluster=w7098) -> (array=w7106:string[])
          }
          frame "UCB Fleezers 052511" {
            w7188 = 2  # Channel pattern
            n1395 = Decimate 1D Array(w7151) -> (w7186:i16[], w7185:i16[], w7150:i16[], w7149:i16[], w7143:i16[], w7140:i16[], w7139:i16[], w7138:i16[])
            n1396 = Decimate 1D Array(w7186) -> (w7184:i16[], w7169:i16[])
            n1397 = Decimate 1D Array(w7185) -> (w7183:i16[], w7181:i16[])
            n1398 = Decimate 1D Array(w7150) -> (w7182:i16[], w7180:i16[])
            n1399 = Decimate 1D Array(w7149) -> (w7145:i16[], w7144:i16[])
            n1400 = Decimate 1D Array(w7143) -> (w7142:i16[], w7141:i16[])
            n1401 = call "downsample 1D array - I16.vi"("Ave N"=2.0, "Array In"=w7140) -> ("Array Out"=w7137:i16[])  [unwired: 1 in]
            n1402 = call "downsample 1D array - I16.vi"("Ave N"=2.0, "Array In"=w7139) -> ("Array Out"=w7136:i16[])  [unwired: 1 in]
            n1403 = call "downsample 1D array - I16.vi"("Ave N"=2.0, "Array In"=w7138) -> ("Array Out"=w7135:i16[])  [unwired: 1 in]
            n1404 = Interleave 1D Arrays(w7184, w7183, w7182, w7169, w7181, w7180, w7145, w7142, w7144, w7141, w7137, w7136, w7135) -> (w7146:i16[])
            n1405 = Divide(x=w7146, y=3276.7) -> (x/y=w7176:dbl[])
            n1406 = Decimate 1D Array(w7176) -> (w7175:dbl[], w7174:dbl[], w7173:dbl[], w7172:dbl[], w7171:dbl[], w7170:dbl[], w7134:dbl[], w7132:dbl[], w7131:dbl[], w7129:dbl[], w7128:dbl[], w7127:dbl[], w7126:dbl[])
            n1407 = Divide(x=w7175, y=w7173) -> (x/y=w7156:dbl[])
            n1408 = Divide(x=w7174, y=w7173) -> (x/y=w7155:dbl[])
            n1409 = Divide(x=w7172, y=w7170) -> (x/y=w7154:dbl[])
            n1410 = Divide(x=w7171, y=w7170) -> (x/y=w7153:dbl[])
            n1411 = Divide(x=w7134, y=w7132) -> (x/y=w7133:dbl[])
            n1412 = Divide(x=w7131, y=w7129) -> (x/y=w7130:dbl[])
            n1413 = Bundle("T1 Y", "T1 X", "T1 Sum", "T2 Y", "T2 X", "T2 Sum", "T1 FB X", "T2 FB Sum", "T2 FB X", "T2 FB Sum", "PSD Y", "PSD X", "PSD Sum") -> (w7157:T46)  [unwired: 1 out]
            n1414 = Build Array(w7156, w7155, w7173, w7154, w7153, w7170, w7133, w7132, w7130, w7129, w7128, w7127, w7126) -> (w7125:dbl[][])
            n1415 = Cluster To Array(cluster=w7157) -> (array=w7148:string[])
          }
          frame "IR-QPD + PSD + FB-QPD XY positions" {
            w7234 = 4  # Channel pattern
            # "time average x2 the 3 psd signals (detection laser)"
            # "deinterlace 3 signals from qpds"
            n1416 = Decimate 1D Array(w7258) -> (w7257:i16[], w7256:i16[], w7235:i16[], w7255:i16[], w7201:i16[], w7247:i16[], w7246:i16[], w7223:i16[])
            n1417 = Decimate 1D Array "QPD Y"(w7257) -> (w7254:i16[], w7237:i16[])
            n1418 = call "downsample 1D array - double.vi"("Ave N"=2.0, "Array In"=w7247) -> ("Array Out"=w7222:dbl[])  [unwired: 1 out]
            n1419 = call "downsample 1D array - double.vi"("Ave N"=2.0, "Array In"=w7246) -> ("Array Out"=w7221:dbl[])  [unwired: 1 out]
            n1420 = Decimate 1D Array "Feedback Sum"(w7235) -> (w7219:i16[], w7217:i16[])
            n1421 = Decimate 1D Array "Feedback Y"(w7201) -> (w7200:i16[], w7199:i16[])
            n1422 = Decimate 1D Array "Feedback X"(w7223) -> (w7220:i16[], w7218:i16[])
            n1423 = Decimate 1D Array "QPD Sum"(w7255) -> (w7252:i16[], w7250:i16[])
            n1424 = Decimate 1D Array "QPD X"(w7256) -> (w7253:i16[], w7251:i16[])
            n1425 = Interleave 1D Arrays(w7254, w7253, w7252, w7237, w7251, w7250, w7200, w7220, w7219, w7199, w7218, w7217, w7222, w7221) -> (w7245:dbl[])
            n1426 = To Word Integer(number=w7245) -> (16bit integer=w7189:i16[])
            n1427 = Divide(x=w7245, y=3276.7) -> (x/y=w7244:dbl[])
            n1428 = Decimate 1D Array(w7244) -> (w7243:dbl[], w7242:dbl[], w7241:dbl[], w7240:dbl[], w7239:dbl[], w7238:dbl[], w7196:dbl[], w7210:dbl[], w7194:dbl[], w7195:dbl[], w7208:dbl[], w7192:dbl[], w7206:dbl[], w7204:dbl[])
            n1429 = Divide(x=w7243, y=w7241) -> (x/y=w7227:dbl[])
            n1430 = Divide(x=w7242, y=w7241) -> (x/y=w7226:dbl[])
            n1431 = Divide(x=w7240, y=w7238) -> (x/y=w7225:dbl[])
            n1432 = Divide(x=w7239, y=w7238) -> (x/y=w7224:dbl[])
            n1433 = Divide(x=w7196, y=w7194) -> (x/y=w7193:dbl[])
            n1434 = Divide(x=w7210, y=w7194) -> (x/y=w7209:dbl[])
            n1435 = Divide(x=w7195, y=w7192) -> (x/y=w7191:dbl[])
            n1436 = Divide(x=w7208, y=w7192) -> (x/y=w7207:dbl[])
            n1437 = Negate(x=w7204) -> (-x=w7202:dbl[])
            n1438 = Divide(x=w7206, y=w7202) -> (x/y=w7205:dbl[])
            n1439 = Bundle("T1 Y", "T1 X", "T1 Sum", "T2 Y", "T2 X", "T2 Sum", "T1 FB Y", "T1 FB X", "T1 FB Sum", "T2 FB Y", "T2 FB X", "T2 FB Sum", "PSD X", "PSD Y Sum") -> (w7190:T47)  [unwired: 1 out]
            n1440 = Build Array(w7227, w7226, w7241, w7225, w7224, w7238, w7193, w7209, w7194, w7191, w7207, w7192, w7205, w7204) -> (w7203:dbl[][])
            n1441 = Cluster To Array(cluster=w7190) -> (array=w7236:string[])
          }
        }
      }
    }
    "AI labels" <- w5527
    n1442 = Decimate 1D Array(w5497) -> (w5525:u32[], w5461:u32[])
    n1443 = local read "DMA Update Period (s)"() -> (w5536:dbl)
    n1444 = local read "BD 1 Frequency 2 (MHz)"() -> (w5403:dbl)
    n1445 = local read "BD 1 Frequency 1 (MHz)"() -> (w5404:dbl)
    n1446 = Build Array(w5525, w5461) -> (w5604:u32[][])
    n1447 = local read "Data Period (s)"() -> (w5510:dbl)
    n1448 = Decimate 1D Array(w5411) -> (w5434:i16[], w5433:i16[], w5431:i16[], w5430:i16[])  [unwired: 9 out]
    n1449 = To Double Precision Float(number=w5604) -> (double precision float=w5605:dbl[][])
    n1450 = local read "APD Integration Time (s)"() -> (w5474:dbl)
    n1451 = Divide(x=w5434, y=w5433) -> (x/y=w5435:dbl[])
    n1452 = Divide(x=w5431, y=w5430) -> (x/y=w5432:dbl[])
    n1453 = feedback #1(0.0) -> (w5448:dbl)
    n1454 = Add(x=w5536, y=w5448) -> (x+y=w5644:dbl)
    n1455 = feedback-in #1(w5644) -> ()
    n1456 = local read "AOM X Cal (nm/MHz)"() -> (w5401:dbl)
    n1457 = To Time Stamp(1:w5448) -> (0:w5447:timestamp)
    n1458 = Split 1D Array(array=w5435, index="N El. to Ave.") -> (second subarray=w5438:dbl[])  [unwired: 1 out]
    n1459 = Split 1D Array(array=w5432, index="N El. to Ave.") -> (second subarray=w5437:dbl[])  [unwired: 1 out]
    n1460 = local read "Trap X AI1 (DMA)"() -> (w5436:T13)
    n1461 = Multiply(x=w5510, y="Trap Disp. Downsample") -> (x*y=w5449:dbl)
    "Display Period (s)" <- w5449
    n1462 = Bundle("BD 1 Frequency 1 (MHz)"=w5404, "BD 1 Frequency 2 (MHz)"=w5403) -> (w5405:T48)  [unwired: 1 out]
    n1463 = for "Trap AI" {
      tunnel: [w6924] -> w5638 mode=indexing
      tunnel: w5447 -> [w6914]
      tunnel: "Trap Disp. Downsample" -> [w6922]
      tunnel: w5528 -> [w6920] mode=indexing
      tunnel: w5510 -> [w6919]
      tunnel: w5527 -> [w6918] mode=indexing
      tunnel: w5446 -> [w6917]
      tunnel: [w6916] -> w5485 mode=indexing
      tunnel: w5449 -> [w6915]
      n1464 = Bundle By Name("Y"=w6920, "dt"=w6919) -> (w6921:waveform(dbl))  [unwired: 1 out]
      n1465 = Set Waveform Attribute(5:w6918, 6:w6917, 7:w6921) -> (3:w6916:waveform(dbl))  [unwired: 1 in, 2 out]
      n1466 = call "downsample 1D array - double.vi"("Ave N"=w6922, "Array In"=w6920) -> ("Array Out"=w6923:dbl[])  [unwired: 1 out]
      n1467 = Bundle By Name(cluster=w6916, "t0"=w6914, "Y"=w6923, "dt"=w6915) -> (w6924:waveform(dbl))
    }
    n1468 = call <vilib>:"Mean.vi"("X"=w5437) -> ("mean"=w5425:dbl)  [unwired: 1 out]
    n1469 = call <vilib>:"Mean.vi"("X"=w5438) -> ("mean"=w5426:dbl)  [unwired: 1 out]
    n1470 = Cluster To Array(cluster=w5405) -> (array=w5402:dbl[])
    n1471 = Reciprocal(x=w5449) -> (1/x=→"Trap Disp. Freq. (Hz)":dbl)
    n1472 = local read "Data points/scans (MCL)"() -> (w5616:dbl)
    n1473 = To Fixed-Point(number=w5425) -> (fixed-point=w5423:fxp<+/-,16,1>)  [unwired: 1 in]
    n1474 = To Fixed-Point(number=w5426) -> (fixed-point=w5424:fxp<+/-,16,1>)  [unwired: 1 in]
    n1475 = Bundle("Trap 1 Pos.", "Trap 2 Pos.") -> (w5445:cluster{string, string})  [unwired: 1 out]
    n1476 = Bundle By Name(cluster=w5436, "Set 1"=w5424, "Set 2"=w5423) -> (→"Trap X AI1 (DMA)":T13)
    n1477 = Cluster To Array(cluster=w5445) -> (array=w5442:string[])
    n1478 = for "Trap Position" {
      tunnel: w5451 -> [w5901] mode=indexing
      tunnel: "Trap Disp. Downsample" -> [w5900]
      tunnel: w5449 -> [w5898]
      tunnel: w5447 -> [w5897]
      tunnel: w5446 -> [w5895]
      tunnel: w5442 -> [w5894] mode=indexing
      tunnel: [w5893] -> w5400 mode=indexing
      tunnel: w5402 -> [w5891] mode=indexing
      tunnel: w5401 -> [w5889]
      n1479 = call "downsample 1D array - double.vi"("Ave N"=w5900, "Array In"=w5901) -> ("Array Out"=w5899:dbl[])  [unwired: 1 out]
      n1480 = Subtract(x=w5899, y=w5891) -> (x-y=w5892:dbl[])
      n1481 = Multiply(x=w5889, y=w5892) -> (x*y=w5890:dbl[])
      n1482 = Bundle By Name("Y"=w5890, "dt"=w5898, "t0"=w5897) -> (w5896:waveform(dbl))  [unwired: 1 out]
      n1483 = Set Waveform Attribute(5:w5894, 6:w5895, 7:w5896) -> (3:w5893:waveform(dbl))  [unwired: 1 in, 2 out]
    }
    "Trap Positions" <- w5400
    n1484 = Bundle("APD 1", "APD 2") -> (w5637:cluster{string, string})  [unwired: 1 out]
    n1485 = Cluster To Array(cluster=w5637) -> (array=w5634:string[])
    n1486 = for "APD" {
      tunnel: w5605 -> [w6903] mode=indexing
      tunnel: w5474 -> [w6911]
      tunnel: [w6907] -> w5481 mode=indexing
      tunnel: "APD Disp. Scale" -> [w6908]
      tunnel: w5446 -> [w6906]
      tunnel: w5634 -> [w6905] mode=indexing
      tunnel: "APD Disp. Downsample" -> [w6901]
      tunnel: [w6904] -> w5633
      tunnel: w5447 -> [w6900]
      n1487 = call "integrate 1D array interval - double.vi"("Ave N"=w6901, "Array In"=w6903) -> ("Array Out"=w6902:dbl[])  [unwired: 1 out]
      n1488 = Multiply(x=w6911, y=w6901) -> (x*y=w6904:dbl)
      n1489 = Divide(x=w6902, y=w6908) -> (x/y=w6909:dbl[])
      n1490 = Bundle By Name("t0"=w6900, "Y"=w6909, "dt"=w6904) -> (w6910:waveform(dbl))  [unwired: 1 out]
      n1491 = Set Waveform Attribute(5:w6905, 6:w6906, 7:w6910) -> (3:w6907:waveform(dbl))  [unwired: 1 in, 2 out]
    }
    "APD Display Period (s)" <- w5633
    n1492 = Reciprocal(x=w5633) -> (1/x=→"APD Display Freq. (Hz)":dbl)
    n1493 = local read "Display Period (s)"() -> (w5509:dbl)
    n1494 = Increment(x=w5616) -> (x+1=w5617:dbl)
    n1495 = Index Array(array=w5400, index=0) -> (element=w5398:waveform(dbl))
    n1496 = To Double Precision Float(number=w5525) -> (double precision float=w5524:dbl[])
    n1497 = feedback #2(w5617) -> (w5620:dbl)
    n1498 = Select(t=0, s=w5607, f=w5620) -> (s? t:f=w5613:dbl)
    n1499 = Array Size(array=w5524) -> (size(s)=w5619:i32)
    n1500 = Add(x=w5619, y=w5613) -> (x+y=w5614:dbl)
    n1501 = Unbundle By Name(w5398) -> ("Y"=w5396:dbl[])
    n1502 = feedback #3(w5525) -> (w5603:u32[])
    n1503 = Build Array (concatenate)(w5603, w5525) -> (w5600:u32[])
    n1504 = feedback #4(w5461) -> (w5480:u32[])
    n1505 = Divide(x="Bead Sep. Int. Time (s)", y=w5509) -> (x/y=w5394:dbl)
    n1506 = Build Array (concatenate)(w5480, w5461) -> (w5479:u32[])
    n1507 = Greater?(x=w5614, y=w5616) -> (0:w5615:bool)
    n1508 = feedback #5(w5396) -> (w5397:dbl[])
    n1509 = Build Array (concatenate)(w5396, w5397) -> (w5395:dbl[])
    n1510 = Select(t=w5613, s=w5615, f=w5614) -> (s? t:f=w5612:dbl)
    n1511 = feedback-in #2(w5612) -> ()
    n1512 = Array Size(array=w5600) -> (size(s)=w5597:i32)
    n1513 = Array Size(array=w5525) -> (size(s)=w5599:i32)
    n1514 = local read "MCL Scanning"() -> (w5610:bool)
    n1515 = local read "APD Integration Time (s)"() -> (w5488:dbl)
    n1516 = Build Array (concatenate)(w5481, w5638) -> (w5483:waveform(dbl)[])
    "All Signals" <- w5483
    n1517 = Split 1D Array(array=w5395, index=w5394) -> (first subarray=w5388:dbl[])  [unwired: 1 out]
    n1518 = feedback-in #5(w5388) -> ()
    n1519 = Multiply(x=w5599, y="APD Ave N") -> (x*y=w5598:dbl)
    n1520 = Greater?(x=w5597, y=w5598) -> (0:w5601:bool)
    n1521 = Not(x=w5615) -> (.not. x?=w5609:bool)
    n1522 = To Double Precision Float(number=w5461) -> (double precision float=w5460:dbl[])
    n1523 = call <vilib>:"Mean.vi"("X"=w5388) -> ("mean"=w5387:dbl)  [unwired: 1 out]
    "Mean T1 Position (nm)" <- w5387
    n1524 = Subtract(x=w5388, y=w5387) -> (x-y=w5393:dbl[])
    n1525 = Square(x=w5393) -> (x^2=w5392:dbl[])
    n1526 = And(x=w5609, y=w5610) -> (x .and. y?=w5611:bool)
    n1527 = call <vilib>:"Mean.vi"("X"=w5392) -> ("mean"=w5391:dbl)  [unwired: 1 out]
    n1528 = case shown="True" w5601 {
      tunnel: w5600 -> [w6484 w6491]
      tunnel: [w6484 w6489] -> w5541
      tunnel: w5598 -> [_ w6486]
      tunnel: w5597 -> [_ w6490]